vi "Dresden R2R Sputter 03.02.2018 IY24.vi"() -> ()   [LabVIEW 2009] (continued)
                                }
                                frame #1 {
                                }
                                }
                                }
                                }
                              }
                              frame #1 {
                              }
                            }
                          }
                          frame #14 {
                            # "CLOSE CH-VBV"
                            n19975 = local read "Semi"() -> (w24598:bool)
                            n19976 = case shown="False" w24598 {
                              frame #0 {
                                n19977 = stacked-sequence {
                                frame #0 {
                                n19978 = local read "Semi"() -> (w24599:bool)
                                n19979 = case shown="False" w24599 {
                                frame #0 {
                                n19980 = while {
                                i -> [w24606]
                                stop <- w24600 stop-if-true
                                n19981 = Greater?(x=w24606, y=50) -> (0:w24604:bool)
                                n19982 = case shown="True" w24604 {
                                frame #0 {
                                }
                                frame #1 {
                                n19983 = local write "Semi"(TRUE ("Semi")) -> ()
                                n19984 = local write "Error Message"("Start up process  cancelled\nbecause  CH-VBV not closed.\nPlease check  CH3-VBV connections." ("Error Message")) -> ()
                                }
                                }
                                n19985 = local read "Ch3_Ch_vbv_di"() -> (w24603:bool)
                                n19986 = case shown="True" w24603 {
                                tunnel: [TRUE FALSE] -> w24602
                                frame #0 {
                                }
                                frame #1 {
                                n19987 = Wait Until Next ms Multiple(millisecond multiple=u32 200) -> ()  [unwired: 1 out]
                                n19988 = local write "Ch3_Ch_vbv_do"(FALSE ("Ch1_Tp_bv_do")) -> ()
                                }
                                }
                                n19989 = local read "Semi"() -> (w24601:bool)
                                n19990 = Or(x=w24602, y=w24601) -> (x .or. y?=w24600:bool)
                                }
                                }
                                frame #1 {
                                }
                                }
                                }
                                frame #1 {
                                n19991 = local read "Semi"() -> (w24613:bool)
                                n19992 = case shown="False" w24613 {
                                frame #0 {
                                n19993 = local write "Ch3_PA20"(TRUE ("PA3")) -> ()
                                n19994 = Wait Until Next ms Multiple(millisecond multiple=u32 1000) -> ()  [unwired: 1 out]
                                }
                                frame #1 {
                                }
                                }
                                }
                                }
                              }
                              frame #1 {
                              }
                            }
                          }
                          frame #15 {
                            # "Close PL-VBV"
                            n19995 = local read "Semi"() -> (w24616:bool)
                            n19996 = case shown="False" w24616 {
                              frame #0 {
                                n19997 = stacked-sequence {
                                frame #0 {
                                n19998 = local read "Semi"() -> (w24617:bool)
                                n19999 = case shown="False" w24617 {
                                frame #0 {
                                n20000 = while {
                                i -> [w24624]
                                stop <- w24618 stop-if-true
                                n20001 = Greater?(x=w24624, y=50) -> (0:w24622:bool)
                                n20002 = case shown="True" w24622 {
                                frame #0 {
                                }
                                frame #1 {
                                n20003 = local write "Semi"(TRUE ("Semi")) -> ()
                                n20004 = local write "Error Message"("Start up process  cancelled\nbecause  PL-VBV not closed.\nPlease check PL3-VBV connections." ("Error Message")) -> ()
                                }
                                }
                                n20005 = local read "Ch3_Pl_vbv_di"() -> (w24621:bool)
                                n20006 = case shown="True" w24621 {
                                tunnel: [TRUE FALSE] -> w24620
                                frame #0 {
                                }
                                frame #1 {
                                n20007 = Wait Until Next ms Multiple(millisecond multiple=u32 200) -> ()  [unwired: 1 out]
                                n20008 = local write "Ch3_Pl_vbv_do"(FALSE ("Ch1_Tp_bv_do")) -> ()
                                }
                                }
                                n20009 = local read "Semi"() -> (w24619:bool)
                                n20010 = Or(x=w24620, y=w24619) -> (x .or. y?=w24618:bool)
                                }
                                }
                                frame #1 {
                                }
                                }
                                }
                                frame #1 {
                                n20011 = local read "Semi"() -> (w24631:bool)
                                n20012 = case shown="False" w24631 {
                                frame #0 {
                                n20013 = local write "Ch3_PA21"(TRUE ("PA3")) -> ()
                                n20014 = Wait Until Next ms Multiple(millisecond multiple=u32 1000) -> ()  [unwired: 1 out]
                                }
                                frame #1 {
                                }
                                }
                                }
                                }
                              }
                              frame #1 {
                              }
                            }
                          }
                          frame #16 {
                            # "OPEN TP-BV"
                            n20015 = local read "Semi"() -> (w24634:bool)
                            n20016 = case shown="False" w24634 {
                              frame #0 {
                                n20017 = stacked-sequence {
                                frame #0 {
                                n20018 = local read "Semi"() -> (w24635:bool)
                                n20019 = case shown="False" w24635 {
                                frame #0 {
                                n20020 = while {
                                i -> [w24642]
                                stop <- w24637 stop-if-true
                                n20021 = Greater?(x=w24642, y=50) -> (0:w24640:bool)
                                n20022 = case shown="True" w24640 {
                                frame #0 {
                                }
                                frame #1 {
                                n20023 = local write "Semi"(TRUE ("Semi")) -> ()
                                n20024 = local write "Error Message"("Start up process  cancelled\nbecause  TP-BV not opened.\nPlease check TP-BV3 connections." ("Error Message")) -> ()
                                }
                                }
                                n20025 = local read "Ch3_Tp_bv_di"() -> (w24636:bool)
                                n20026 = case shown="False" w24636 {
                                tunnel: [FALSE TRUE] -> w24639
                                frame #0 {
                                n20027 = Wait Until Next ms Multiple(millisecond multiple=u32 200) -> ()  [unwired: 1 out]
                                n20028 = local write "Ch3_Tp_bv_do"(TRUE ("Ch1_Tp_bv_do")) -> ()
                                }
                                frame #1 {
                                }
                                }
                                n20029 = local read "Semi"() -> (w24638:bool)
                                n20030 = Or(x=w24639, y=w24638) -> (x .or. y?=w24637:bool)
                                }
                                }
                                frame #1 {
                                }
                                }
                                }
                                frame #1 {
                                n20031 = local read "Semi"() -> (w24649:bool)
                                n20032 = case shown="False" w24649 {
                                frame #0 {
                                n20033 = local write "Ch3_PA22"(TRUE ("PA3")) -> ()
                                n20034 = Wait Until Next ms Multiple(millisecond multiple=u32 1000) -> ()  [unwired: 1 out]
                                }
                                frame #1 {
                                }
                                }
                                }
                                }
                              }
                              frame #1 {
                              }
                            }
                          }
                          frame #17 {
                            # "CLOSE CH-ATM"
                            n20035 = local read "Semi"() -> (w24652:bool)
                            n20036 = case shown="False" w24652 {
                              frame #0 {
                                n20037 = stacked-sequence {
                                frame #0 {
                                n20038 = local read "Semi"() -> (w24653:bool)
                                n20039 = case shown="False" w24653 {
                                frame #0 {
                                n20040 = while {
                                i -> [w24660]
                                stop <- w24654 stop-if-true
                                n20041 = Greater?(x=w24660, y=50) -> (0:w24658:bool)
                                n20042 = case shown="True" w24658 {
                                frame #0 {
                                }
                                frame #1 {
                                n20043 = local write "Semi"(TRUE ("Semi")) -> ()
                                n20044 = local write "Error Message"("Start up process  cancelled\nbecause CH-ATM not closed.\nPlease check CH3-ATM connections." ("Error Message")) -> ()
                                }
                                }
                                n20045 = local read "Ch3_Ch_atm_di"() -> (w24657:bool)
                                n20046 = case shown="True" w24657 {
                                tunnel: [TRUE FALSE] -> w24656
                                frame #0 {
                                }
                                frame #1 {
                                n20047 = Wait Until Next ms Multiple(millisecond multiple=u32 200) -> ()  [unwired: 1 out]
                                n20048 = local write "Ch3_Ch_atm_do"(TRUE ("Ch1_Tp_bv_do")) -> ()
                                }
                                }
                                n20049 = local read "Semi"() -> (w24655:bool)
                                n20050 = Or(x=w24656, y=w24655) -> (x .or. y?=w24654:bool)
                                }
                                }
                                frame #1 {
                                }
                                }
                                }
                                frame #1 {
                                n20051 = local read "Semi"() -> (w24667:bool)
                                n20052 = case shown="False" w24667 {
                                frame #0 {
                                n20053 = local write "Ch3_PA23"(TRUE ("PA3")) -> ()
                                n20054 = Wait Until Next ms Multiple(millisecond multiple=u32 1000) -> ()  [unwired: 1 out]
                                }
                                frame #1 {
                                }
                                }
                                }
                                }
                              }
                              frame #1 {
                              }
                            }
                          }
                          frame #18 {
                            # "CLOSE PL-ATM"
                            n20055 = local read "Semi"() -> (w24670:bool)
                            n20056 = case shown="False" w24670 {
                              frame #0 {
                                n20057 = stacked-sequence {
                                frame #0 {
                                n20058 = local read "Semi"() -> (w24671:bool)
                                n20059 = case shown="False" w24671 {
                                frame #0 {
                                n20060 = while {
                                i -> [w24678]
                                stop <- w24672 stop-if-true
                                n20061 = Greater?(x=w24678, y=50) -> (0:w24676:bool)
                                n20062 = case shown="True" w24676 {
                                frame #0 {
                                }
                                frame #1 {
                                n20063 = local write "Semi"(TRUE ("Semi")) -> ()
                                n20064 = local write "Error Message"("Start up process  cancelled\nbecause  PL-ATM not closed.\nPlease check PL-ATM3 connections." ("Error Message")) -> ()
                                }
                                }
                                n20065 = local read "Ch3_Pl_atm_di"() -> (w24675:bool)
                                n20066 = case shown="True" w24675 {
                                tunnel: [TRUE FALSE] -> w24674
                                frame #0 {
                                }
                                frame #1 {
                                n20067 = Wait Until Next ms Multiple(millisecond multiple=u32 200) -> ()  [unwired: 1 out]
                                n20068 = local write "Ch3_Pl_atm_do"(TRUE ("Ch1_Tp_bv_do")) -> ()
                                }
                                }
                                n20069 = local read "Semi"() -> (w24673:bool)
                                n20070 = Or(x=w24674, y=w24673) -> (x .or. y?=w24672:bool)
                                }
                                }
                                frame #1 {
                                }
                                }
                                }
                                frame #1 {
                                n20071 = local read "Semi"() -> (w24685:bool)
                                n20072 = case shown="False" w24685 {
                                frame #0 {
                                n20073 = local write "Ch3_PA24"(TRUE ("PA3")) -> ()
                                n20074 = Wait Until Next ms Multiple(millisecond multiple=u32 1000) -> ()  [unwired: 1 out]
                                }
                                frame #1 {
                                }
                                }
                                }
                                }
                              }
                              frame #1 {
                              }
                            }
                          }
                          frame #19 {
                            # "START MP"
                            n20075 = local read "Semi"() -> (w24688:bool)
                            n20076 = case shown="False" w24688 {
                              frame #0 {
                                n20077 = stacked-sequence {
                                frame #0 {
                                n20078 = local read "Semi"() -> (w24689:bool)
                                n20079 = case shown="False" w24689 {
                                frame #0 {
                                n20080 = while {
                                i -> [w24696]
                                stop <- w24690 stop-if-true
                                n20081 = Greater?(x=w24696, y=50) -> (0:w24694:bool)
                                n20082 = case shown="True" w24694 {
                                frame #0 {
                                }
                                frame #1 {
                                n20083 = local write "Semi"(TRUE ("Semi")) -> ()
                                n20084 = local write "Error Message"("Start up process  cancelled\nbecause MP not started.\nPlease check MP3 connections." ("Error Message")) -> ()
                                }
                                }
                                n20085 = local read "Ch3_Mp_di"() -> (w24693:bool)
                                n20086 = case shown="False" w24693 {
                                tunnel: [FALSE TRUE] -> w24692
                                frame #0 {
                                n20087 = Wait Until Next ms Multiple(millisecond multiple=u32 200) -> ()  [unwired: 1 out]
                                n20088 = local write "Ch3_Mp_do"(TRUE ("Ch1_Tp_bv_do")) -> ()
                                }
                                frame #1 {
                                }
                                }
                                n20089 = local read "Semi"() -> (w24691:bool)
                                n20090 = Or(x=w24692, y=w24691) -> (x .or. y?=w24690:bool)
                                }
                                }
                                frame #1 {
                                }
                                }
                                }
                                frame #1 {
                                n20091 = local read "Semi"() -> (w24703:bool)
                                n20092 = case shown="False" w24703 {
                                frame #0 {
                                n20093 = local write "Ch3_PA25"(TRUE ("PA3")) -> ()
                                n20094 = Wait Until Next ms Multiple(millisecond multiple=u32 1000) -> ()  [unwired: 1 out]
                                }
                                frame #1 {
                                }
                                }
                                }
                                }
                              }
                              frame #1 {
                              }
                            }
                          }
                          frame #20 {
                            # "START TP"
                            n20095 = local read "Semi"() -> (w24706:bool)
                            n20096 = case shown="False" w24706 {
                              frame #0 {
                                n20097 = stacked-sequence {
                                frame #0 {
                                n20098 = local read "Semi"() -> (w24707:bool)
                                n20099 = case shown="False" w24707 {
                                frame #0 {
                                n20100 = stacked-sequence {
                                frame #0 {
                                n20101 = local read "Semi"() -> (w24708:bool)
                                n20102 = case shown="False" w24708 {
                                frame #0 {
                                n20103 = local write "Tp3_auto_start"(TRUE ("Tp1_auto_start")) -> ()
                                }
                                frame #1 {
                                }
                                }
                                }
                                frame #1 {
                                n20104 = local read "Semi"() -> (w24710:bool)
                                n20105 = case shown="False" w24710 {
                                frame #0 {
                                n20106 = Wait (ms)(milliseconds to wait=u32 1000) -> ()  [unwired: 1 out]
                                }
                                frame #1 {
                                }
                                }
                                }
                                frame #2 {
                                n20107 = local read "Semi"() -> (w24712:bool)
                                n20108 = case shown="False" w24712 {
                                frame #0 {
                                n20109 = local write "Tp3_auto_start"(TRUE ("Tp1_auto_start")) -> ()
                                }
                                frame #1 {
                                }
                                }
                                }
                                }
                                }
                                frame #1 {
                                }
                                }
                                }
                                frame #1 {
                                n20110 = local read "Semi"() -> (w24714:bool)
                                n20111 = case shown="False" w24714 {
                                frame #0 {
                                n20112 = local write "Ch3_PA30"(TRUE ("PA3")) -> ()
                                n20113 = Wait Until Next ms Multiple(millisecond multiple=u32 1000) -> ()  [unwired: 1 out]
                                }
                                frame #1 {
                                }
                                }
                                }
                                }
                              }
                              frame #1 {
                              }
                            }
                          }
                          frame #21 {
                            # "CHECK PL-PRESSURE"
                            n20114 = local read "Semi"() -> (w24717:bool)
                            n20115 = case shown="False" w24717 {
                              frame #0 {
                                n20116 = stacked-sequence {
                                frame #0 {
                                n20117 = local read "Semi"() -> (w24718:bool)
                                n20118 = case shown="False" w24718 {
                                frame #0 {
                                n20119 = while {
                                i -> [w24727]
                                stop <- w24722 stop-if-true
                                n20120 = Greater?(x=w24727, y=1200) -> (0:w24725:bool)
                                n20121 = case shown="True" w24725 {
                                frame #0 {
                                }
                                frame #1 {
                                n20122 = local write "Semi"(TRUE ("Semi")) -> ()
                                n20123 = local write "Error Message"("Start up process was cancelled.\nPlease check Pipeline \nvacuum connections." ("Error Message")) -> ()
                                }
                                }
                                n20124 = local read "Pl_pg_press_ch3"() -> (w24721:dbl)
                                n20125 = Less?(x=w24721, y=0.9) -> (x < y?=w24719:bool)
                                n20126 = case shown="False" w24719 {
                                tunnel: [FALSE TRUE] -> w24724
                                frame #0 {
                                n20127 = Wait Until Next ms Multiple(millisecond multiple=u32 500) -> ()  [unwired: 1 out]
                                }
                                frame #1 {
                                }
                                }
                                n20128 = local read "Semi"() -> (w24723:bool)
                                n20129 = Or(x=w24724, y=w24723) -> (x .or. y?=w24722:bool)
                                }
                                }
                                frame #1 {
                                }
                                }
                                }
                                frame #1 {
                                n20130 = local read "Semi"() -> (w24733:bool)
                                n20131 = case shown="False" w24733 {
                                frame #0 {
                                n20132 = local write "Ch3_PA26"(TRUE ("PA3")) -> ()
                                n20133 = Wait Until Next ms Multiple(millisecond multiple=u32 1000) -> ()  [unwired: 1 out]
                                }
                                frame #1 {
                                }
                                }
                                }
                                }
                              }
                              frame #1 {
                              }
                            }
                          }
                          frame #22 {
                            # "CHECK CH-PRESSURE"
                            n20134 = local read "Semi"() -> (w24736:bool)
                            n20135 = case shown="False" w24736 {
                              frame #0 {
                                n20136 = stacked-sequence {
                                frame #0 {
                                n20137 = local read "Semi"() -> (w24737:bool)
                                n20138 = case shown="False" w24737 {
                                frame #0 {
                                n20139 = while {
                                i -> [w24746]
                                stop <- w24741 stop-if-true
                                n20140 = Greater?(x=w24746, y=1200) -> (0:w24744:bool)
                                n20141 = case shown="True" w24744 {
                                frame #0 {
                                }
                                frame #1 {
                                n20142 = local write "Semi"(TRUE ("Semi")) -> ()
                                n20143 = local write "Error Message"("Start up process was cancelled.\nPlease check chamber \nvacuum connections." ("Error Message")) -> ()
                                }
                                }
                                n20144 = local read "Ch3_pressure"() -> (w24740:dbl)
                                n20145 = Less?(x=w24740, y=0.9) -> (x < y?=w24738:bool)
                                n20146 = case shown="False" w24738 {
                                tunnel: [FALSE TRUE] -> w24743
                                frame #0 {
                                n20147 = Wait Until Next ms Multiple(millisecond multiple=u32 500) -> ()  [unwired: 1 out]
                                }
                                frame #1 {
                                }
                                }
                                n20148 = local read "Semi"() -> (w24742:bool)
                                n20149 = Or(x=w24743, y=w24742) -> (x .or. y?=w24741:bool)
                                }
                                }
                                frame #1 {
                                }
                                }
                                }
                                frame #1 {
                                n20150 = local read "Semi"() -> (w24752:bool)
                                n20151 = case shown="False" w24752 {
                                frame #0 {
                                n20152 = local write "Ch3_PA27"(TRUE ("PA3")) -> ()
                                n20153 = Wait Until Next ms Multiple(millisecond multiple=u32 1000) -> ()  [unwired: 1 out]
                                }
                                frame #1 {
                                }
                                }
                                }
                                }
                              }
                              frame #1 {
                              }
                            }
                          }
                          frame #23 {
                            # "OPEN BG-BV"
                            n20154 = local read "Semi"() -> (w24755:bool)
                            n20155 = case shown="False" w24755 {
                              frame #0 {
                                n20156 = stacked-sequence {
                                frame #0 {
                                n20157 = local read "Semi"() -> (w24756:bool)
                                n20158 = case shown="False" w24756 {
                                frame #0 {
                                n20159 = while {
                                i -> [w24763]
                                stop <- w24758 stop-if-true
                                n20160 = Greater?(x=w24763, y=50) -> (0:w24761:bool)
                                n20161 = case shown="True" w24761 {
                                frame #0 {
                                }
                                frame #1 {
                                n20162 = local write "Semi"(TRUE ("Semi")) -> ()
                                n20163 = local write "Error Message"("Start up process  cancelled\nbecause  BG-BV not opened.\nPlease check BG-BV3 connections." ("Error Message")) -> ()
                                }
                                }
                                n20164 = local read "Ch3_Bg_bv_di"() -> (w24757:bool)
                                n20165 = case shown="False" w24757 {
                                tunnel: [FALSE TRUE] -> w24760
                                frame #0 {
                                n20166 = Wait Until Next ms Multiple(millisecond multiple=u32 200) -> ()  [unwired: 1 out]
                                n20167 = local write "Ch3_Bg_bv_do"(TRUE ("Ch1_Tp_bv_do")) -> ()
                                }
                                frame #1 {
                                }
                                }
                                n20168 = local read "Semi"() -> (w24759:bool)
                                n20169 = Or(x=w24760, y=w24759) -> (x .or. y?=w24758:bool)
                                }
                                }
                                frame #1 {
                                }
                                }
                                }
                                frame #1 {
                                n20170 = local read "Semi"() -> (w24770:bool)
                                n20171 = case shown="False" w24770 {
                                frame #0 {
                                n20172 = local write "Ch3_PA28"(TRUE ("PA3")) -> ()
                                n20173 = Wait Until Next ms Multiple(millisecond multiple=u32 1000) -> ()  [unwired: 1 out]
                                }
                                frame #1 {
                                }
                                }
                                }
                                }
                              }
                              frame #1 {
                              }
                            }
                          }
                          frame #24 {
                            # "CHECK CH-PRESSURE"
                            n20174 = local read "Semi"() -> (w24773:bool)
                            n20175 = case shown="False" w24773 {
                              frame #0 {
                                n20176 = stacked-sequence {
                                frame #0 {
                                n20177 = local read "Semi"() -> (w24774:bool)
                                n20178 = case shown="False" w24774 {
                                frame #0 {
                                n20179 = while {
                                i -> [w24783]
                                stop <- w24778 stop-if-true
                                n20180 = Greater?(x=w24783, y=600) -> (0:w24781:bool)
                                n20181 = case shown="True" w24781 {
                                frame #0 {
                                }
                                frame #1 {
                                n20182 = local write "Semi"(TRUE ("Semi")) -> ()
                                n20183 = local write "Error Message"("Start up process was cancelled.\nPlease check chamber \nvacuum connections." ("Error Message")) -> ()
                                }
                                }
                                n20184 = local read "Ch3_pressure"() -> (w24777:dbl)
                                n20185 = Less?(x=w24777, y=0.9) -> (x < y?=w24775:bool)
                                n20186 = case shown="False" w24775 {
                                tunnel: [FALSE TRUE] -> w24780
                                frame #0 {
                                n20187 = Wait Until Next ms Multiple(millisecond multiple=u32 500) -> ()  [unwired: 1 out]
                                }
                                frame #1 {
                                }
                                }
                                n20188 = local read "Semi"() -> (w24779:bool)
                                n20189 = Or(x=w24780, y=w24779) -> (x .or. y?=w24778:bool)
                                }
                                }
                                frame #1 {
                                }
                                }
                                }
                                frame #1 {
                                n20190 = local read "Semi"() -> (w24789:bool)
                                n20191 = case shown="False" w24789 {
                                frame #0 {
                                n20192 = local write "Ch3_PA29"(TRUE ("PA3")) -> ()
                                n20193 = Wait Until Next ms Multiple(millisecond multiple=u32 1000) -> ()  [unwired: 1 out]
                                }
                                frame #1 {
                                }
                                }
                                }
                                }
                              }
                              frame #1 {
                              }
                            }
                          }
                          frame #25 {
                            # "START TP"
                            n20194 = local read "Semi"() -> (w24792:bool)
                            n20195 = case shown="False" w24792 {
                              frame #0 {
                                n20196 = stacked-sequence {
                                frame #0 {
                                n20197 = local read "Semi"() -> (w24793:bool)
                                n20198 = case shown="False" w24793 {
                                frame #0 {
                                n20199 = stacked-sequence {
                                frame #0 {
                                n20200 = local read "Semi"() -> (w24794:bool)
                                n20201 = case shown="False" w24794 {
                                frame #0 {
                                n20202 = local write "Tp3_auto_start"(TRUE ("Tp1_auto_start")) -> ()
                                }
                                frame #1 {
                                }
                                }
                                }
                                frame #1 {
                                n20203 = local read "Semi"() -> (w24796:bool)
                                n20204 = case shown="False" w24796 {
                                frame #0 {
                                n20205 = Wait (ms)(milliseconds to wait=u32 1000) -> ()  [unwired: 1 out]
                                }
                                frame #1 {
                                }
                                }
                                }
                                frame #2 {
                                n20206 = local read "Semi"() -> (w24798:bool)
                                n20207 = case shown="False" w24798 {
                                frame #0 {
                                n20208 = while {
                                i -> [w24804]
                                stop <- w24800 stop-if-true
                                n20209 = local read "TP3_working"() -> (w24802:bool)
                                n20210 = Greater?(x=w24804, y=120) -> (0:w24803:bool)
                                n20211 = local read "Semi"() -> (w24801:bool)
                                n20212 = Compound Arithmetic op=OR(w24801, w24802, w24803) -> (w24800:bool)
                                n20213 = Wait (ms)(milliseconds to wait=u32 500) -> ()  [unwired: 1 out]
                                }
                                }
                                frame #1 {
                                }
                                }
                                }
                                frame #3 {
                                n20214 = local read "Semi"() -> (w24806:bool)
                                n20215 = case shown="False" w24806 {
                                frame #0 {
                                n20216 = local read "TP3_working"() -> (w24807:bool)
                                n20217 = case shown="False" w24807 {
                                frame #0 {
                                n20218 = local write "Tp3_auto_start"(TRUE ("Pc_bv1_auto_open")) -> ()
                                }
                                frame #1 {
                                }
                                }
                                }
                                frame #1 {
                                }
                                }
                                }
                                frame #4 {
                                n20219 = local read "Semi"() -> (w24809:bool)
                                n20220 = case shown="False" w24809 {
                                frame #0 {
                                n20221 = local read "TP3_working"() -> (w24810:bool)
                                n20222 = case shown="False" w24810 {
                                frame #0 {
                                n20223 = Wait (ms)(milliseconds to wait=u32 1000) -> ()  [unwired: 1 out]
                                }
                                frame #1 {
                                }
                                }
                                }
                                frame #1 {
                                }
                                }
                                }
                                frame #5 {
                                n20224 = local read "Semi"() -> (w24812:bool)
                                n20225 = case shown="False" w24812 {
                                frame #0 {
                                n20226 = while {
                                i -> [w24818]
                                stop <- w24814 stop-if-true
                                n20227 = local read "TP3_working"() -> (w24816:bool)
                                n20228 = Greater?(x=w24818, y=120) -> (0:w24817:bool)
                                n20229 = local read "Semi"() -> (w24815:bool)
                                n20230 = Compound Arithmetic op=OR(w24815, w24816, w24817) -> (w24814:bool)
                                n20231 = Wait (ms)(milliseconds to wait=u32 500) -> ()  [unwired: 1 out]
                                }
                                }
                                frame #1 {
                                }
                                }
                                }
                                frame #6 {
                                n20232 = local read "Semi"() -> (w24820:bool)
                                n20233 = case shown="False" w24820 {
                                frame #0 {
                                n20234 = local read "TP3_working"() -> (w24821:bool)
                                n20235 = case shown="False" w24821 {
                                frame #0 {
                                n20236 = local write "Error Message"("Start up process  cancelled\nbecause  TP not started.\nPlease check TP3 connections." ("Error Message")) -> ()
                                n20237 = Wait (ms)(milliseconds to wait=u32 1000) -> ()  [unwired: 1 out]
                                }
                                frame #1 {
                                }
                                }
                                }
                                frame #1 {
                                }
                                }
                                }
                                }
                                }
                                frame #1 {
                                }
                                }
                                }
                                frame #1 {
                                n20238 = local read "Semi"() -> (w24824:bool)
                                n20239 = case shown="False" w24824 {
                                frame #0 {
                                n20240 = local write "Ch3_PA30"(TRUE ("PA3")) -> ()
                                n20241 = Wait Until Next ms Multiple(millisecond multiple=u32 1000) -> ()  [unwired: 1 out]
                                }
                                frame #1 {
                                }
                                }
                                }
                                }
                              }
                              frame #1 {
                              }
                            }
                          }
                          frame #26 {
                            # "CHECK CH-PRESSURE"
                            n20242 = local read "Semi"() -> (w24827:bool)
                            n20243 = case shown="False" w24827 {
                              frame #0 {
                                n20244 = stacked-sequence {
                                frame #0 {
                                n20245 = local read "Semi"() -> (w24828:bool)
                                n20246 = case shown="False" w24828 {
                                frame #0 {
                                n20247 = while {
                                i -> [w24837]
                                stop <- w24832 stop-if-true
                                n20248 = Greater?(x=w24837, y=240) -> (0:w24835:bool)
                                n20249 = case shown="True" w24835 {
                                frame #0 {
                                }
                                frame #1 {
                                n20250 = local write "Semi"(TRUE ("Semi")) -> ()
                                n20251 = local write "Error Message"("Start up process was cancelled.\nPlease check chamber \nvacuum connections." ("Error Message")) -> ()
                                }
                                }
                                n20252 = local read "Ch3_pressure"() -> (w24831:dbl)
                                n20253 = Less?(x=w24831, y=0.9) -> (x < y?=w24829:bool)
                                n20254 = case shown="False" w24829 {
                                tunnel: [FALSE TRUE] -> w24834
                                frame #0 {
                                n20255 = Wait Until Next ms Multiple(millisecond multiple=u32 500) -> ()  [unwired: 1 out]
                                }
                                frame #1 {
                                }
                                }
                                n20256 = local read "Semi"() -> (w24833:bool)
                                n20257 = Or(x=w24834, y=w24833) -> (x .or. y?=w24832:bool)
                                }
                                }
                                frame #1 {
                                }
                                }
                                }
                                frame #1 {
                                n20258 = local read "Semi"() -> (w24843:bool)
                                n20259 = case shown="False" w24843 {
                                frame #0 {
                                n20260 = local write "Ch3_PA31"(TRUE ("PA3")) -> ()